vi "Main - 副本.vi"() -> ()   [LabVIEW 2020]
uses:
  System.Windows.Forms
  Global_Variable/Global.vi
  Database/Global1.vi
  <userlib>/_MGI/Menu Building/MenuTypes/MenuStrip/MGI_MenuStrip.lvclass
  <userlib>/_MGI/Menu Building/MenuItemStatusChange/MGI_MenuItemStatusChange.lvclass
  Libraries/S7/S7.lvlib
panel:
  in  "表格控件 2":string[][](table)
  out "上序状态":string
  out "右工位传感器码":string
  in  "表格控件":string[][](table)
  in  "Andon":enum32{"未选择", "缺料报警", "质量报警", "故障报警"}(radio)
  out "PLC":bool
  in  "菜单":refnum<k24>(container)
  out "试验计时":u16
  out "左工位传感器码":string
  out "生产数量":i32
  out "合格数量":i32
  out "userStatus":string caption="用户状态"
  out "userName":string caption="用户名"
  out "connectionMode":string caption="联机类型"
  out "产品型号":string
  in  "更换产品":refnum<vi>
  out "提示信息":string
  out "错误":bool
  out "时间字符串":string
  out "日期字符串":string
  out "自动":bool
  # "芯轴分总成磨合台"
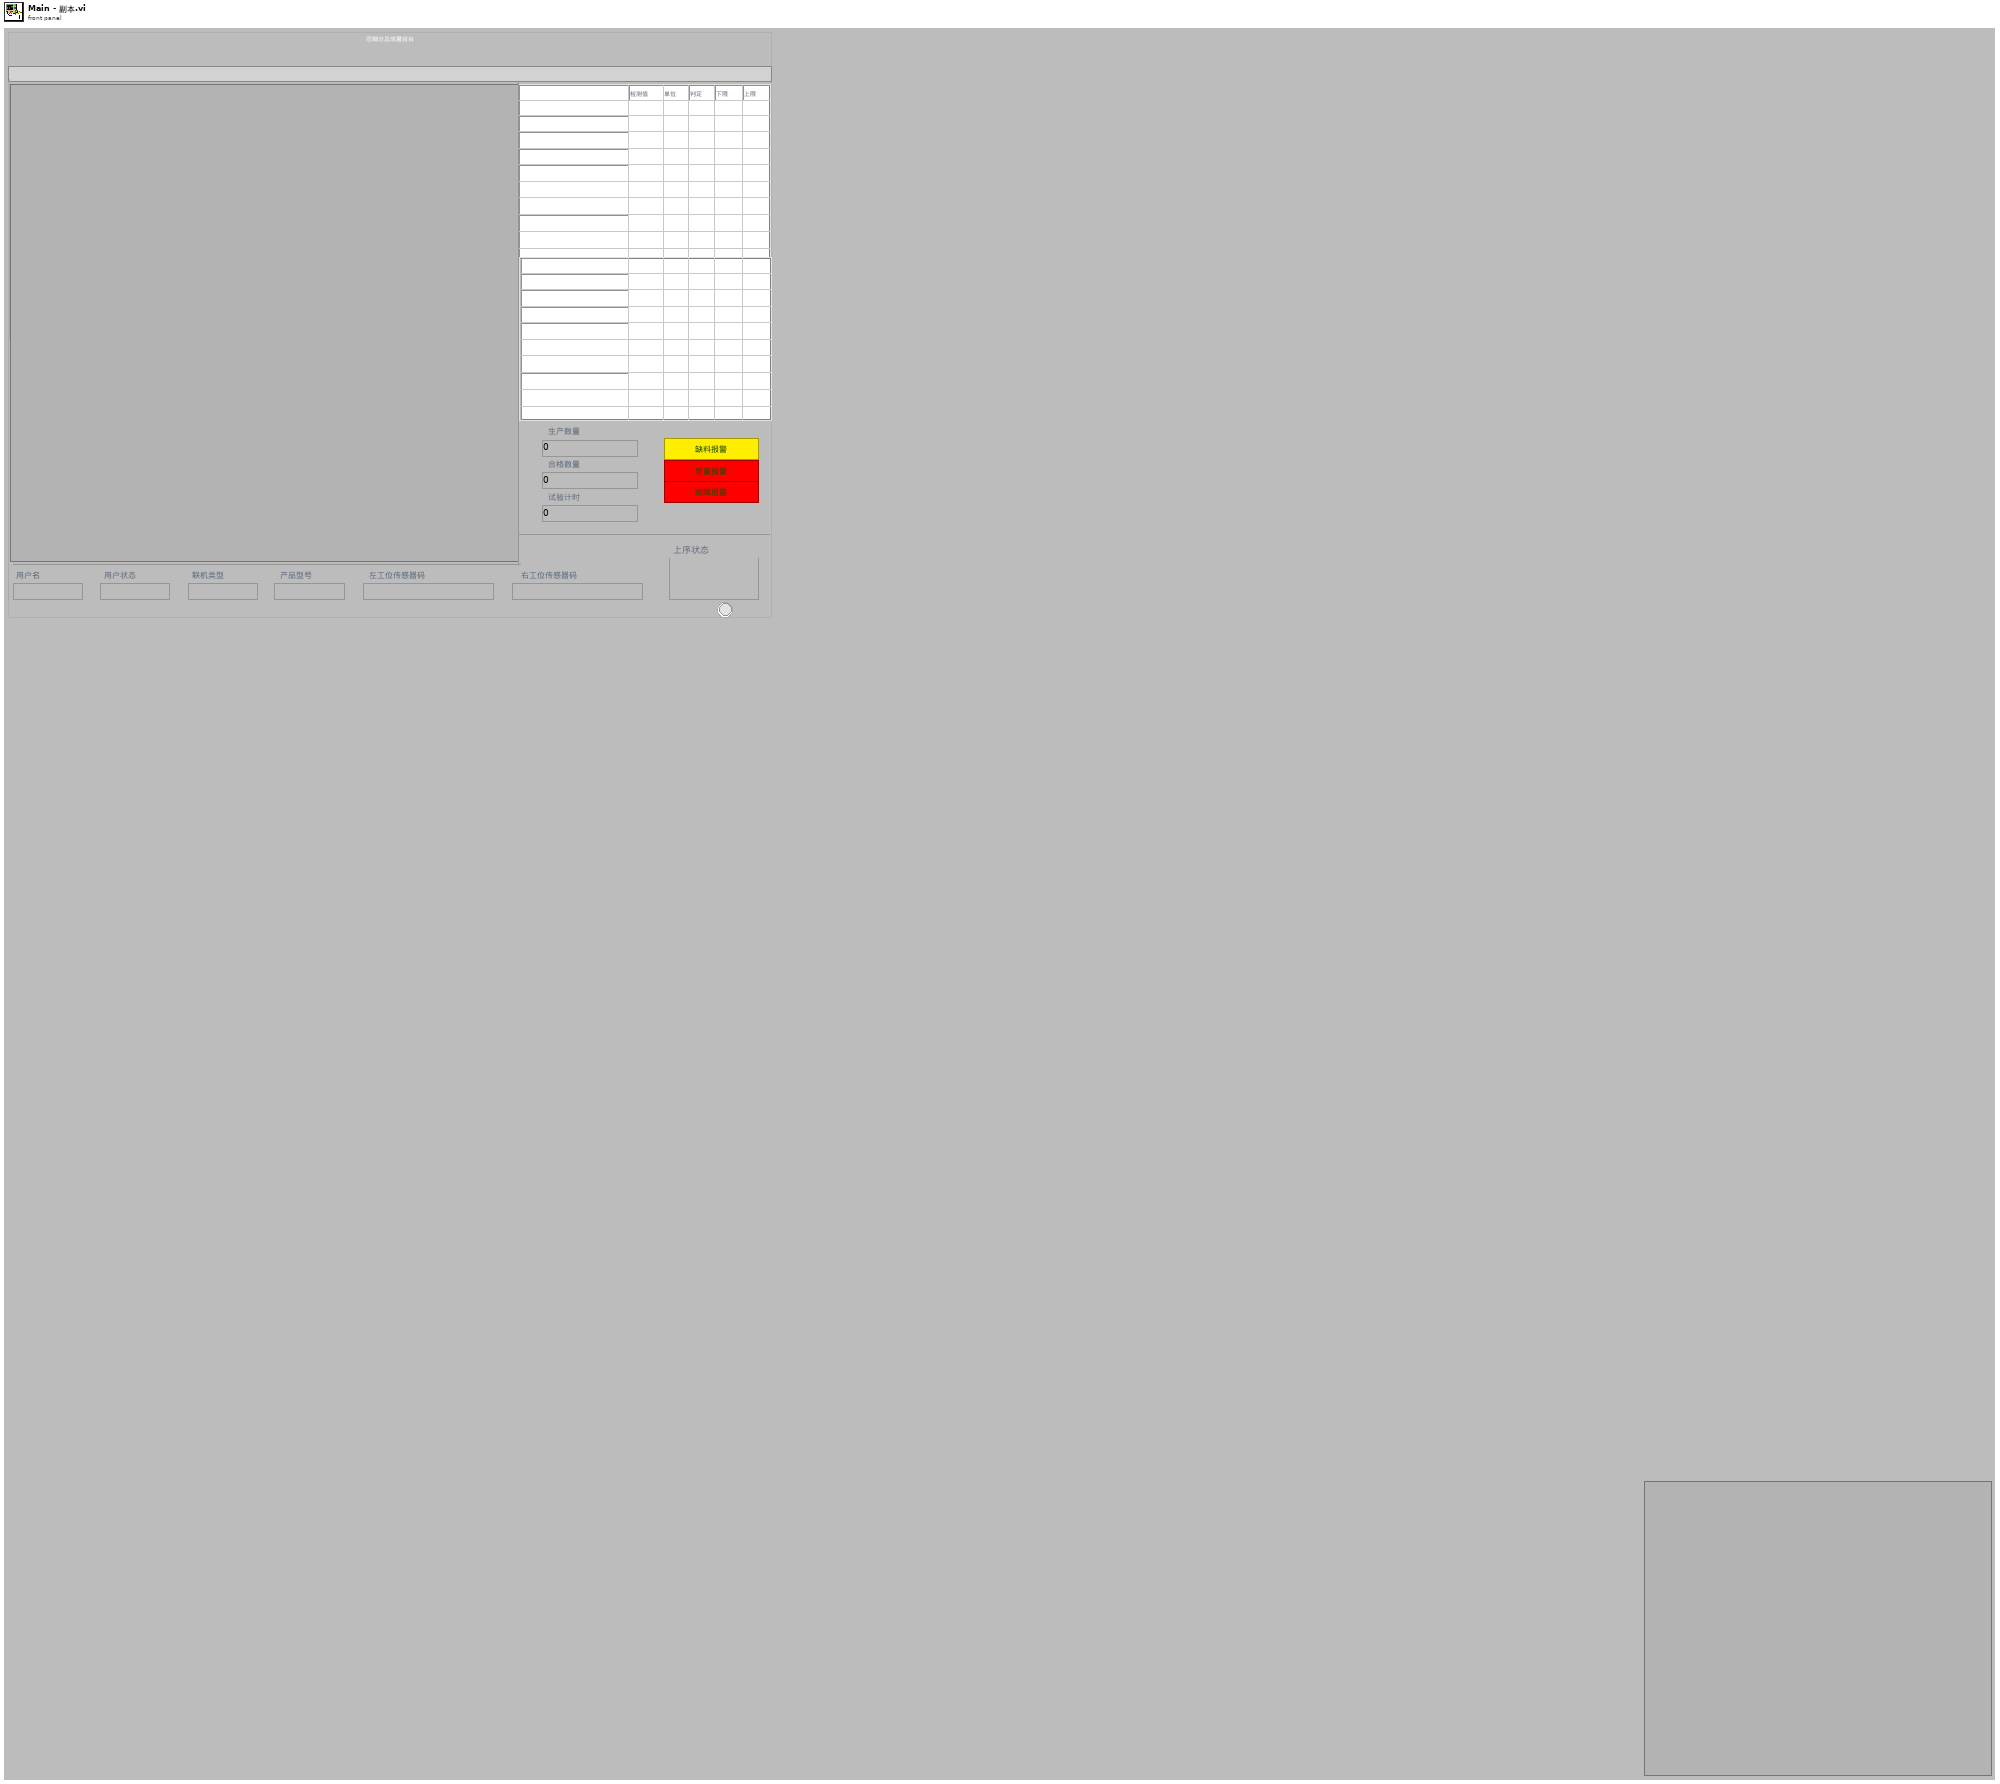
[diagram p1: front panel]
types:
  T1 = typedef "S7.lvlib/Broadcast Events--cluster.ctl" = cluster{"Module Did Init":refnum<user-event>, "Status Updated":refnum<user-event>, "Error Reported":refnum<user-event>, "Module Did Stop":refnum<user-event>, "Update Module Execution Status":refnum<user-event>}
  T2 = enum32{"Invalid", "Standard", "Closed", "Hidden", "Minimized", "Maximized"}
  T3 = cluster{"设备名称":string, "操作人员":string, "设备状态":enum16{"设备离线", "设备正常", "设备缺料", "设备故障", "质量报警"}, "附加信息":string}
  T4 = enum32{"invalid app kind", "Development System", "Run Time System", "Student Edition", "Embedded LabVIEW", "Evaluation", "Custom"}
  T5 = cluster{"用户编号":string, "用户名":string, "用户密码(密文)":string, "用户权限":string}
  T6 = cluster{"Core":cluster{"Current VI Reference":refnum<vi>, "Close Panel on Exit?":bool}, "Your Boolean data":bool, "Your string data":string}
  T7 = cluster{"Current VI Reference":refnum<vi>, "Close Panel on Exit?":bool}
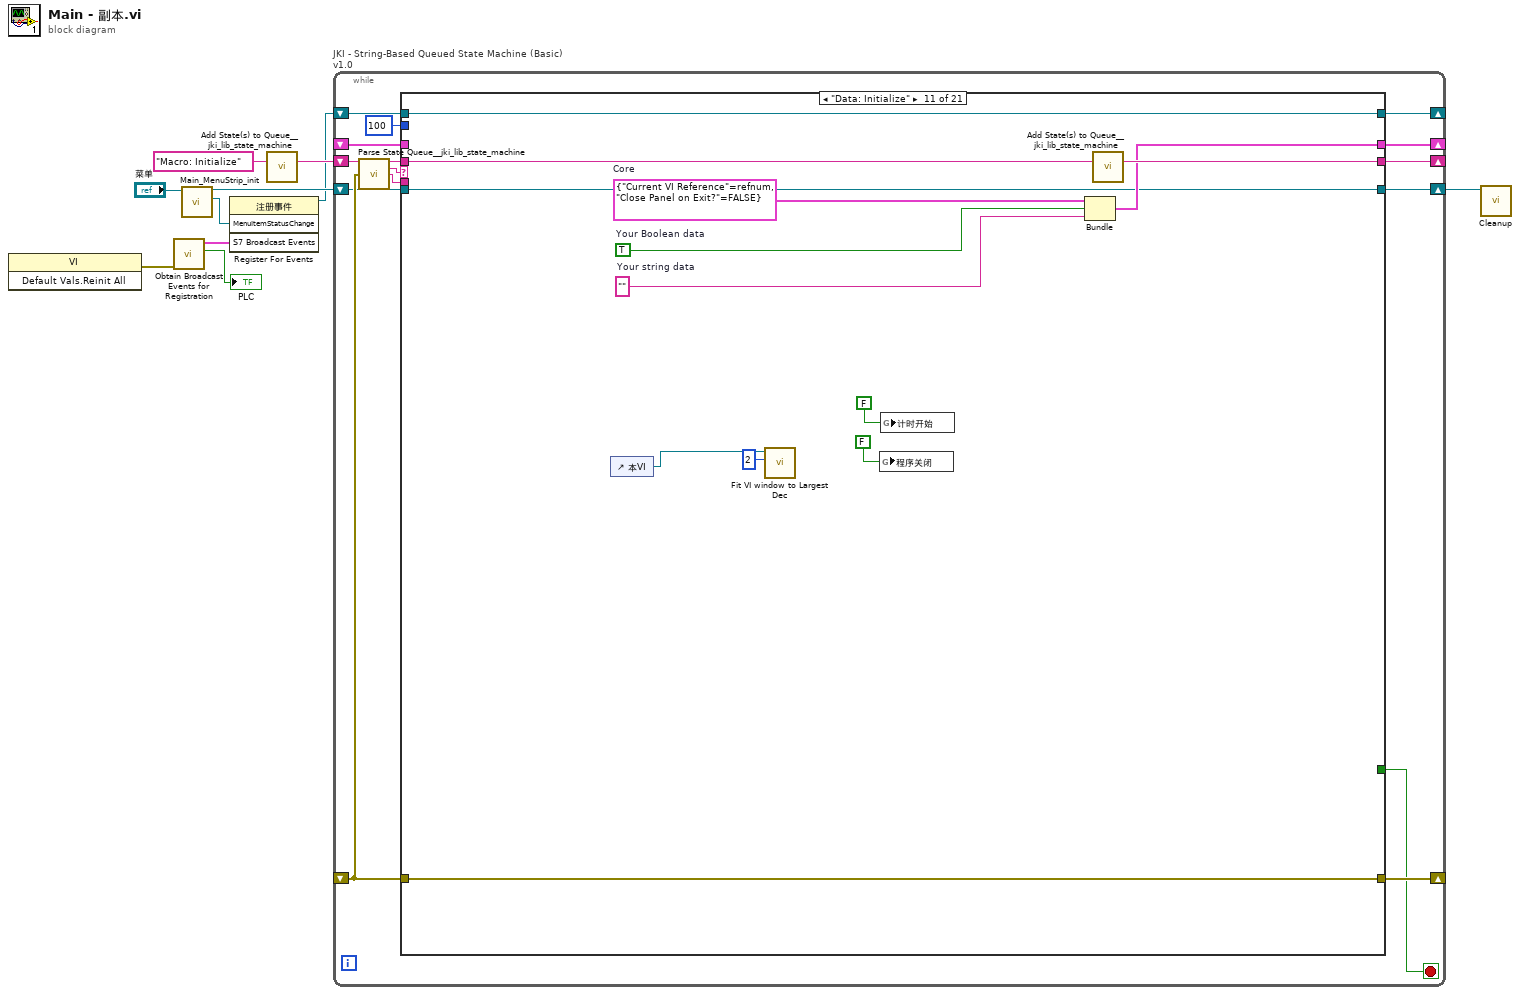
[diagram p0: block diagram]
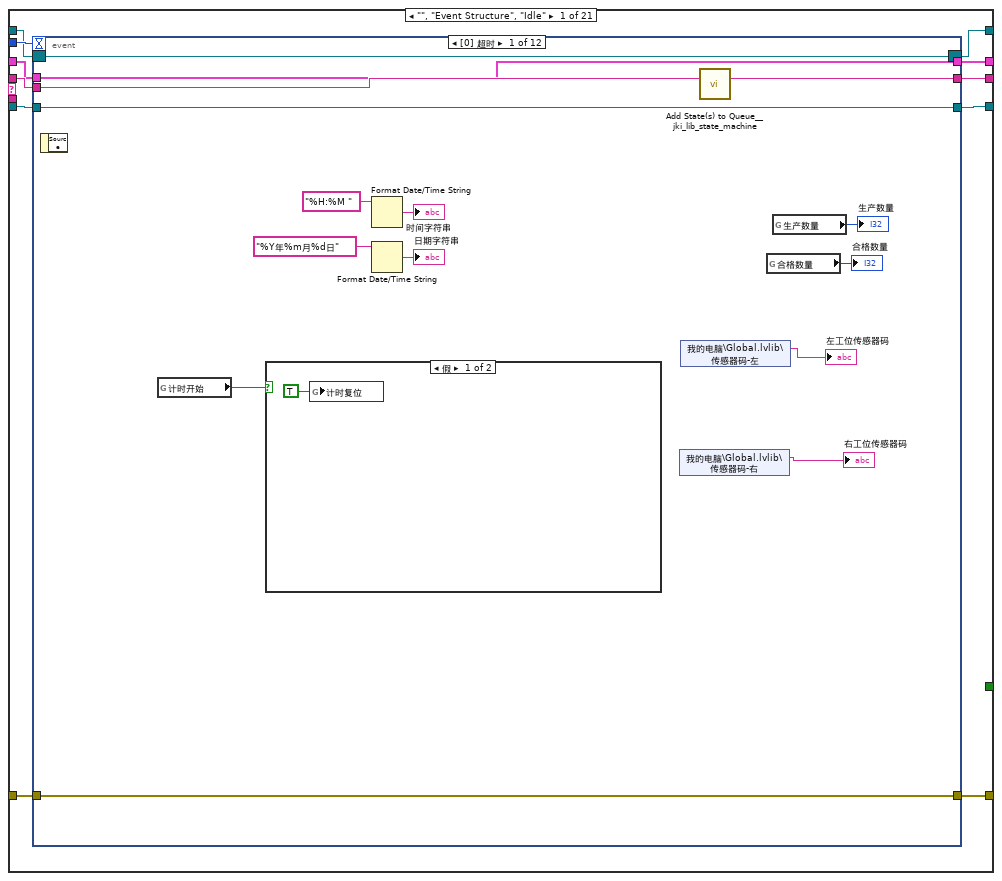
[diagram p2: hidden frame]
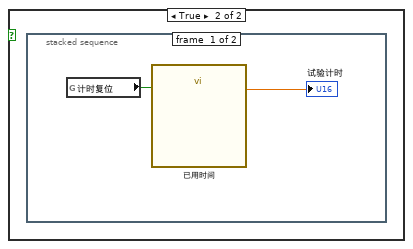
[diagram p3: hidden frame]
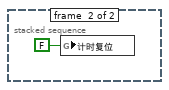
[diagram p4: hidden frame]
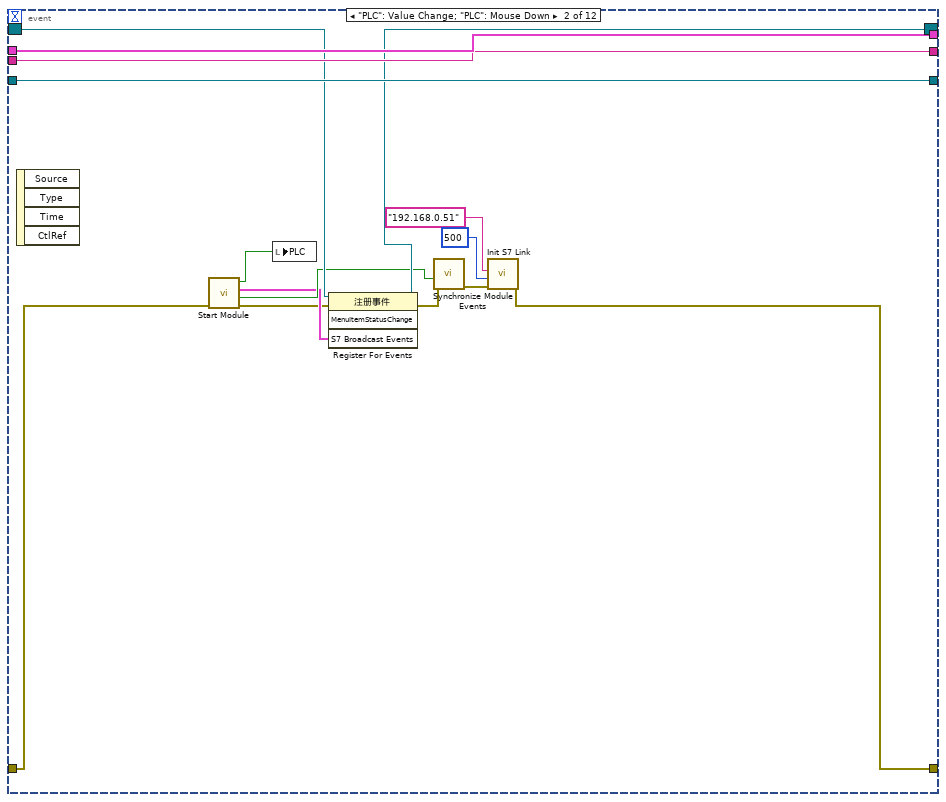
[diagram p5: hidden frame]
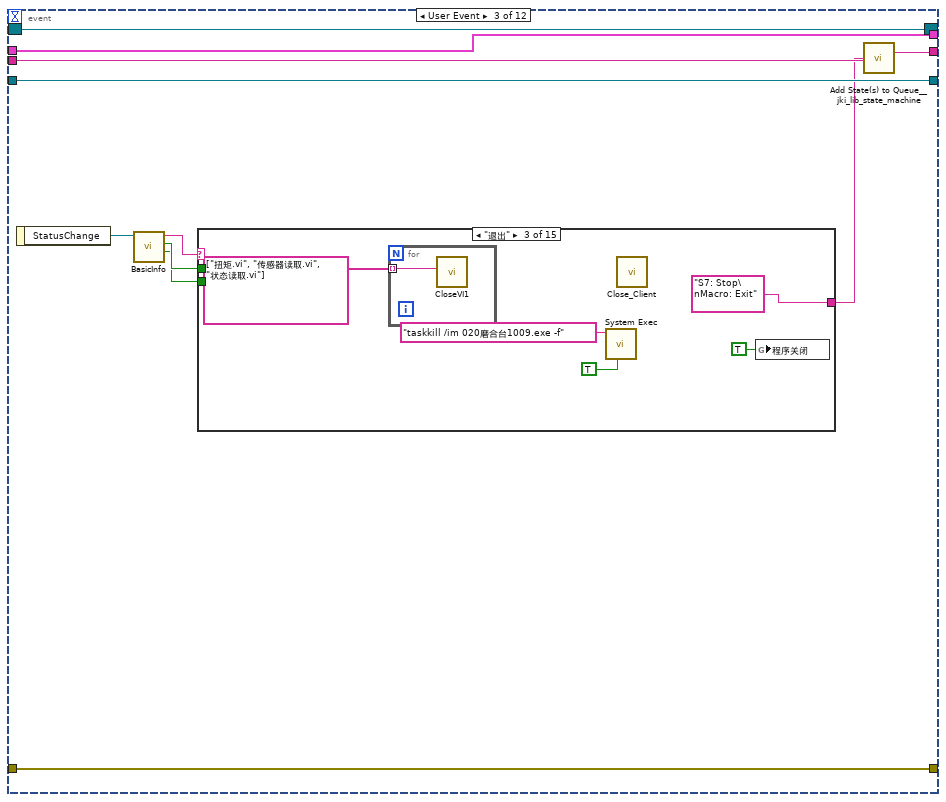
[diagram p6: hidden frame]
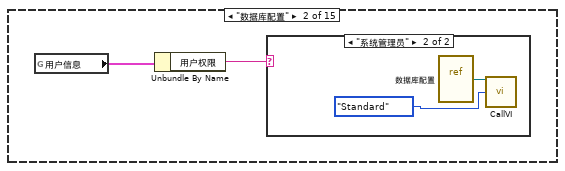
[diagram p8: hidden frame]
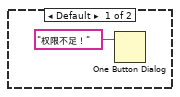
[diagram p9: hidden frame]
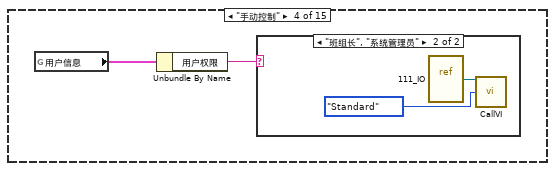
[diagram p10: hidden frame]
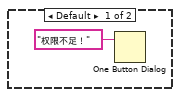
[diagram p11: hidden frame]
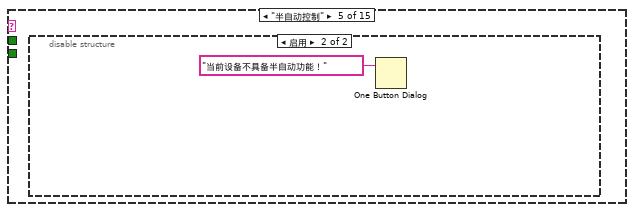
[diagram p12: hidden frame]
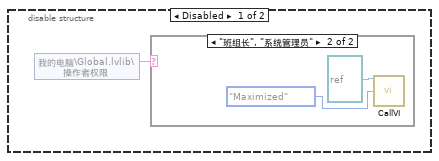
[diagram p13: hidden frame]
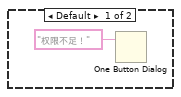
[diagram p14: hidden frame]
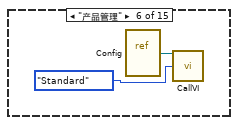
[diagram p15: hidden frame]
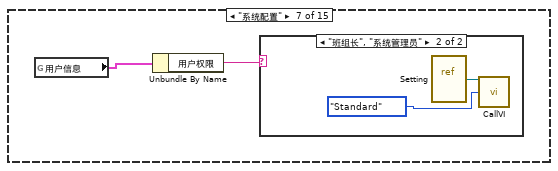
[diagram p16: hidden frame]
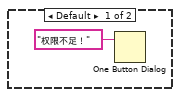
[diagram p17: hidden frame]
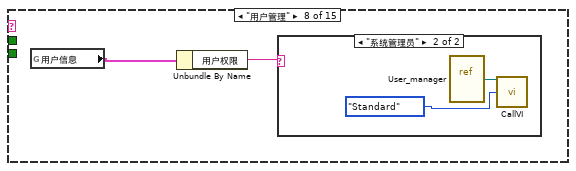
[diagram p18: hidden frame]
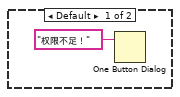
[diagram p19: hidden frame]
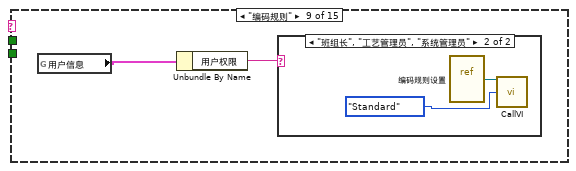
[diagram p20: hidden frame]
diagram:
  n1 = invoke class="VI" method="Default Vals.Reinit All"() -> (error out=w3:errorcluster)  [unwired: 3 in, 2 out]
  n2 = call "Obtain Broadcast Events for Registration.vi"("error in (no error)"=w3) -> ("Already running?"=→"PLC":bool, "S7 Broadcast Events"=w5:T1)  [unwired: 8 in, 1 out]
  n3 = call "Main_MenuStrip_init.vi"("MenuStrip"="菜单") -> ("MenuItemStatusChange"=w2:refnum<user-event>, "Menu out"=w7:refnum<class "MGI_MenuStrip.lvclass">)  [unwired: 9 in]
  n4 = register-events(w2, w5) -> (reference out=w1:refnum<event-registration>)  [unwired: 2 in, 1 out]
  n5 = call <vilib>:"Add State(s) to Queue__jki_lib_state_machine.vi"("State(s) in (\"\")"="Macro: Initialize") -> ("States Out"=w10:string)  [unwired: 14 in]
  n6 = while "JKI - String-Based Queued State Machine (Basic) v1.0" {
    shift-right: [w19] -> _
    shift-left: _ -> [w18]
    shift-right: [w21] -> _
    shift-left: _ -> [w16]
    shift-right: [w20] -> _
    shift-left: w10 -> [w22]
    shift-right: [w14] -> w6
    shift-left: w7 -> [w15]
    shift-right: [w12] -> _
    shift-left: w1 -> [w11]
    stop <- w13 stop-if-true
    n7 = call <vilib>:"Parse State Queue__jki_lib_state_machine.vi"("State Queue"=w22, "Error In (no error)"=w16) -> ("Remaining States"=w24:string, "Current State"=w25:string, "Arguments"=w23:string)  [unwired: 11 in]
    n8 = case shown="\"Data: Initialize\"" w25 {
      selector: w25 -> [_ _ w234 _ _ _ _ _ _ _ _ _ _ _ _ _ _ _ _ _ _]
      tunnel: w24 -> [w36 w231 w238 w258 w266 w274 w280 w284 w290 w299 w312 w320 w326 w339 w363 w400 w408 w421 w449 w456 w468]
      tunnel: w23 -> [_ _ _ _ _ _ _ _ _ _ _ _ _ _ _ _ w403 w415 _ _ _]
      tunnel: w18 -> [w34 w228 w236 w249 w263 w272 w277 w285 w293 w296 _ w315 w323 w337 w361 w397 w406 w417 w446 w453 w465]
      tunnel: [w33 w229 w240 w255 errorcluster {"status"=FALSE, "code"=0, "source"=""} ("error out") w271 w278 w282 w288 w297 w309 w316 w324 w336 w359 w398 w404 w418 w447 w454 w466] -> w21
      tunnel: w16 -> [w32 w229 w239 w255 w262 w271 w278 w282 w289 w297 w309 w317 w324 w333 w359 w398 w405 w419 w447 w454 w466]
      tunnel: [w35 w230 w237 w257 w265 w273 w279 w284 w291 w298 w311 w319 w325 w338 w362 w399 w407 w420 w448 w455 w467] -> w20
      tunnel: [w31 w228 w236 w256 w263 w272 w277 w285 w293 w296 w310 w315 w323 w337 w361 w397 w406 w417 w446 w453 w465] -> w19
      tunnel: 100 ("Timeout") -> [w30 _ _ _ _ _ _ _ _ _ _ _ _ _ _ _ _ _ _ _ _]
      tunnel: w15 -> [w29 w227 w233 w246 w260 w270 w276 w283 w292 w295 w304 w314 w322 w335 w360 w396 w402 w414 w445 w451 w458]
      tunnel: [w28 w227 w233 w246 w260 w270 w276 w283 w292 w295 w304 w314 w322 w335 w360 w396 w402 w414 w445 w451 w458] -> w14
      tunnel: [_ _ _ _ _ TRUE _ _ _ _ _ _ _ _ _ _ _ _ _ _ _] -> w13
      tunnel: [w26 w226 w232 w245 w259 w268 w275 w286 w287 w294 w305 w313 w321 w334 w358 w393 w401 w413 w444 w450 w457] -> w12
      tunnel: w11 -> [w27 w226 w232 w245 w259 w268 w275 w286 w287 w294 w305 w313 w321 w334 w358 w393 w401 w413 w444 w450 w457]
      frame "", "Event Structure", "Idle" {
        n9 = event shown="[0] 超时" {
          selector: w27 -> [w41 w65 w71 w141 w148 w155 w162 w176 w185 w193 w202 _]
          dyn-events: [w41 w64 w71 w141 w148 w155 w162 w176 w185 w193 w202 _] -> w26
          timeout: w30 -> [_ _ _ _ _ _ _ _ _ _ _ _]
          tunnel: w36 -> [w51 w69 w80 w142 w149 w158 w165 w173 w189 w200 w204 w220]
          tunnel: [w50 w69 w78 w143 w150 w159 w166 w174 w190 w199 w205 w220] -> w35
          tunnel: w34 -> [w49 w70 w79 w145 w153 w160 w167 w175 w191 w197 w207 w221]
          tunnel: [w42 w66 w81 w146 w151 w156 w168 w171 w188 w198 w206 w218] -> w33
          tunnel: w32 -> [w42 w67 w81 w146 w151 w156 w169 w171 w188 w198 w206 w218]
          tunnel: [w49 w70 w79 w145 w153 w160 w167 w175 w191 w197 w207 w221] -> w31
          tunnel: w29 -> [w40 w68 w74 w144 w152 w157 w164 w172 _ _ _ w219]
          tunnel: [w40 w68 w74 w144 w152 w157 w164 w172 _ _ _ w219] -> w28
          event Timeout {
            n10 = event-data() -> ()  [unwired: 1 in, 1 out]
            n11 = global read "Global.vi" "计时开始"() -> (w39:bool)
            n12 = case shown="假" w39 {
              frame False {
                n13 = global write "Global.vi" "计时复位"(TRUE ("计时复位")) -> ()
              }
              frame True {
                n14 = stacked-sequence {
                  frame #0 {
                    n15 = global read "Global.vi" "计时复位"() -> (w53:bool)
                    n16 = call "已用时间"("Reset"=w53) -> ("Elapsed Time (s)"=→"试验计时":dbl)  [unwired: 11 in, 7 out]
                  }
                  frame #1 {
                    n17 = global write "Global.vi" "计时复位"(FALSE ("计时复位")) -> ()
                  }
                }
              }
            }
            n18 = Format Date/Time String(time format string (%c)="%H:%M ") -> (date/time string=→"时间字符串":string)  [unwired: 2 in]
            n19 = Format Date/Time String(time format string (%c)="%Y年%m月%d日") -> (date/time string=→"日期字符串":string)  [unwired: 2 in]
            n20 = shared-variable "我的电脑\\Global.lvlib\\传感器码-右"() -> (→"右工位传感器码":string)  [unwired: 1 in, 1 out]
            n21 = shared-variable "我的电脑\\Global.lvlib\\传感器码-左"() -> (→"左工位传感器码":string)  [unwired: 1 in, 1 out]
            n22 = call <vilib>:"Add State(s) to Queue__jki_lib_state_machine.vi"("State(s) in (\"\")"=w51) -> ("States Out"=w50:string)  [unwired: 14 in]
            n23 = global read "Global.vi" "合格数量"() -> (→"合格数量":i32)
            n24 = global read "Global.vi" "生产数量"() -> (→"生产数量":i32)
          }
          event "PLC": Value Change; "PLC": Mouse Down {
            n25 = event-data() -> ()  [unwired: 1 in, 4 out]
            n26 = call "Start Module.vi"("error in (no error)"=w67) -> ("error out"=w60:errorcluster, "Wait for Event Sync?"=w63:bool, "S7 Broadcast Events"=w62:T1, "Module Was Already Running?"=w61:bool)  [unwired: 7 in]
            n27 = local write "PLC"(w61) -> ()
            n28 = register-events(reference=w65, error in=w60, w62) -> (reference out=w64:refnum<event-registration>, error out=w59:errorcluster)  [unwired: 1 in]
            n29 = call "Synchronize Module Events.vi"("error in (no error)"=w59, "Wait for Event Sync?"=w63) -> ("error out"=w56:errorcluster)  [unwired: 9 in]
            n30 = call "Init S7 Link.vi"("error in (no error)"=w56, "超时"=500, "IP"="192.168.0.51") -> ("error out"=w66:errorcluster)  [unwired: 8 in]
          }
          event User Event {
            n31 = event-data() -> ("StatusChange"=w72:refnum<class "MGI_MenuItemStatusChange.lvclass">)  [unwired: 1 in]
            n32 = call <userlib>:"BasicInfo.vi"("MGI_MenuItemStatusChange in"=w72) -> ("Enabled?"=w75:bool, "Checked?"=w76:bool, "Tag"=w77:string)  [unwired: 7 in, 1 out]
            n33 = case shown="\"退出\"" w77 {
              tunnel: w76 -> [_ _ _ _ _ _ _ _ _ _ _ _ _ _ _]
              tunnel: w75 -> [_ _ _ _ _ _ _ _ _ _ _ _ _ _ _]
              tunnel: [_ _ "S7: Stop\nMacro: Exit" _ _ _ _ _ _ _ _ _ _ _ _] -> w73
              frame "假", Default {
              }
              frame "数据库配置" {
                n34 = global read "Global1.vi" "用户信息"() -> (w82:T5)
                n35 = Unbundle By Name(w82) -> ("用户权限"=w83:string)
                n36 = case shown="\"系统管理员\"" w83 {
                  frame Default {
                    n37 = One Button Dialog(message="权限不足！" ("消息")) -> ()  [unwired: 1 in, 1 out]
                  }
                  frame "系统管理员" {
                    n38 = vi-ref "数据库配置.vi"() -> (w86:refnum<vi>)
                    n39 = call "CallVI.vi"("VI引用"=w86, "状态"=T2."Standard") -> ()  [unwired: 11 in, 3 out]
                  }
                }
              }
              frame "退出" {
                n40 = for {
                  tunnel: string[] ["扭矩.vi", "传感器读取.vi", "状态读取.vi"] -> [w92] mode=indexing
                  n41 = call "CloseVI1.vi"("名称或相对路径"=w92) -> ()  [unwired: 10 in, 1 out]
                }
                n42 = call <vilib>:"System Exec.vi"("run minimized? (F)"=TRUE, "command line"="taskkill /im 020磨合台1009.exe -f") -> ()  [unwired: 6 in, 4 out]
                n43 = call "Close_Client.vi"() -> ()  [unwired: 12 in]
                n44 = global write "Global.vi" "程序关闭"(TRUE ("程序关闭")) -> ()
              }
              frame "手动控制" {
                n45 = global read "Global1.vi" "用户信息"() -> (w93:T5)
                n46 = Unbundle By Name(w93) -> ("用户权限"=w94:string)
                n47 = case shown="\"班组长\", \"系统管理员\"" w94 {
                  frame Default {
                    n48 = One Button Dialog(message="权限不足！" ("消息")) -> ()  [unwired: 1 in, 1 out]
                  }
                  frame "班组长", "系统管理员" {
                    n49 = vi-ref "111_IO.vi"() -> (w97:refnum<vi>)
                    n50 = call "CallVI.vi"("VI引用"=w97, "状态"=T2."Standard") -> ()  [unwired: 11 in, 3 out]
                  }
                }
              }
              frame "半自动控制" {
                n51 = disable-structure shown="启用" {
                  frame Disabled {
                    n52 = shared-variable "我的电脑\\Global.lvlib\\操作者权限"() -> (w98:string)  [unwired: 1 in, 1 out]
                    n53 = case shown="\"班组长\", \"系统管理员\"" w98 {
                      frame Default {
                        n54 = One Button Dialog(message="权限不足！" ("消息")) -> ()  [unwired: 1 in, 1 out]
                      }
                      frame "班组长", "系统管理员" {
                        n55 = call "CallVI.vi"("VI引用"=refnum<vi> refnum, "状态"=T2."Maximized") -> ()  [unwired: 11 in, 3 out]
                      }
                    }
                  }
                  frame Enabled {
                    n56 = One Button Dialog(message="当前设备不具备半自动功能！" ("消息")) -> ()  [unwired: 1 in, 1 out]
                  }
                }
              }
              frame "产品管理" {
                n57 = vi-ref "Config.vi"() -> (w104:refnum<vi>)
                n58 = call "CallVI.vi"("VI引用"=w104, "状态"=T2."Standard") -> ()  [unwired: 11 in, 3 out]
              }
              frame "系统配置" {
                n59 = global read "Global1.vi" "用户信息"() -> (w105:T5)
                n60 = Unbundle By Name(w105) -> ("用户权限"=w106:string)
                n61 = case shown="\"班组长\", \"系统管理员\"" w106 {
                  frame Default {
                    n62 = One Button Dialog(message="权限不足！" ("消息")) -> ()  [unwired: 1 in, 1 out]
                  }
                  frame "班组长", "系统管理员" {
                    n63 = vi-ref "Setting.vi"() -> (w109:refnum<vi>)
                    n64 = call "CallVI.vi"("VI引用"=w109, "状态"=T2."Standard") -> ()  [unwired: 11 in, 3 out]
                  }
                }
              }
              frame "用户管理" {
                n65 = global read "Global1.vi" "用户信息"() -> (w110:T5)
                n66 = Unbundle By Name(w110) -> ("用户权限"=w111:string)
                n67 = case shown="\"系统管理员\"" w111 {
                  frame Default {
                    n68 = One Button Dialog(message="权限不足！" ("消息")) -> ()  [unwired: 1 in, 1 out]
                  }
                  frame "系统管理员" {
                    n69 = vi-ref "User_manager.vi"() -> (w114:refnum<vi>)
                    n70 = call "CallVI.vi"("VI引用"=w114, "状态"=T2."Standard") -> ()  [unwired: 11 in, 3 out]
                  }
                }
              }
              frame "编码规则" {
                n71 = global read "Global1.vi" "用户信息"() -> (w115:T5)
                n72 = Unbundle By Name(w115) -> ("用户权限"=w116:string)
                n73 = case shown="\"班组长\", \"工艺管理员\", \"系统管理员\"" w116 {
                  frame Default {
                    n74 = One Button Dialog(message="权限不足！" ("消息")) -> ()  [unwired: 1 in, 1 out]
                  }
                  frame "班组长", "工艺管理员", "系统管理员" {
                    n75 = vi-ref "编码规则设置.vi"() -> (w119:refnum<vi>)
                    n76 = call "CallVI.vi"("VI引用"=w119, "状态"=T2."Standard") -> ()  [unwired: 11 in, 3 out]
                  }
                }
              }
              frame "易损件管理" {
                n77 = vi-ref "易损件管理.vi"() -> (w121:refnum<vi>)
                n78 = call "CallVI.vi"("VI引用"=w121, "状态"=T2."Standard") -> ()  [unwired: 11 in, 3 out]
              }
              frame "物料批次管理" {
                n79 = vi-ref "批次管理.vi"() -> (w123:refnum<vi>)
                n80 = call "CallVI.vi"("VI引用"=w123, "状态"=T2."Standard") -> ()  [unwired: 11 in, 3 out]
              }
              frame "报表" {
                n81 = call "文件对话框"("start path"=path "D:/report", "prompt"="打开报表", "pattern (all files)"="*.doc;*.docx", "pattern label"="Word 文档") -> ("selected path"=w124:path, "error out"=w125:errorcluster)  [unwired: 8 in, 2 out]
                n82 = case shown="无错误" w125 {
                  selector: w125 -> [w131 w133]
                  tunnel: w124 -> [w132 _]
                  frame No Error {
                    w130 = 1 items=["Normal", "Maximize", "Minimize"] ("cpubbs_WindowState")
                    n83 = call "Open_Word.vi"("File Path"=w132, "cpubbs_WindowState"=w130, "错误输入（无错误）"=w131) -> ()  [unwired: 12 in, 1 out]
                  }
                  frame Error {
                    n84 = call <vilib>:"Clear Errors.vi"("error in (no error)"=w133) -> ()  [unwired: 5 in, 2 out]
                  }
                }
              }
              frame "报警信息" {
                n85 = vi-ref "报警信息.vi"() -> (w135:refnum<vi>)
                n86 = call "CallVI.vi"("VI引用"=w135, "状态"=T2."Standard") -> ()  [unwired: 11 in, 3 out]
              }
              frame "关于" {
                n87 = vi-ref "About.vi"() -> (w137:refnum<vi>)
                n88 = call "CallVI.vi"("VI引用"=w137, "状态"=T2."Standard") -> ()  [unwired: 11 in, 3 out]
              }
              frame "操作演示" {
                n89 = call <vilib>:"Application Directory.vi"() -> ("Application Directory"=w140:path)
                n90 = Build Path(base path=w140, name or relative path="操作演示" ("名称或相对路径")) -> (appended path=w139:path)
                n91 = call "自动播放ppt.vi"("路径"=w139) -> ()  [unwired: 10 in, 1 out]
              }
            }
            n92 = call <vilib>:"Add State(s) to Queue__jki_lib_state_machine.vi"("State(s) in (\"\")"=w80, "State(s) at Back (\"\")"=w73) -> ("States Out"=w78:string)  [unwired: 13 in]
          }
          event User Event {
            n93 = event-data() -> ("Init?"=w147:bool)  [unwired: 1 in, 1 out]
            n94 = local write "PLC"(w147) -> ()
            n95 = call <vilib>:"Add State(s) to Queue__jki_lib_state_machine.vi"("State(s) in (\"\")"=w142) -> ("States Out"=w143:string)  [unwired: 14 in]
          }
          event User Event {
            n96 = event-data() -> ("Running?"=w154:bool)  [unwired: 1 in]
            n97 = local write "PLC"(w154) -> ()
            n98 = call <vilib>:"Add State(s) to Queue__jki_lib_state_machine.vi"("State(s) in (\"\")"=w149) -> ("States Out"=w150:string)  [unwired: 14 in]
          }
          event User Event {
            n99 = event-data() -> ()  [unwired: 1 in, 7 out]
            n100 = local write "PLC"(FALSE ("PLC")) -> ()
            n101 = call <vilib>:"Add State(s) to Queue__jki_lib_state_machine.vi"("State(s) in (\"\")"=w158) -> ("States Out"=w159:string)  [unwired: 14 in]
          }
          event User Event {
            n102 = event-data() -> ("Error"=w170:errorcluster)  [unwired: 1 in]
            n103 = Merge Errors(w170, w169) -> (w168:errorcluster)
            n104 = call <vilib>:"Add State(s) to Queue__jki_lib_state_machine.vi"("State(s) in Front (\"\")"="S7: Initialize\nIdle", "State(s) in (\"\")"=w165) -> ("States Out"=w166:string)  [unwired: 13 in]
          }
          event "自动": Mouse Down {
            n105 = event-data() -> ()  [unwired: 1 in, 1 out]
            n106 = disable-structure shown="禁用" {
              frame Disabled {
                n107 = local read "自动"() -> (w177:bool)
                n108 = case shown="假" w177 {
                  frame False {
                    n109 = call "设备状态.vi"() -> ("Status_Read"=w178:i16)  [unwired: 11 in]
                    n110 = case shown="5" w178 {
                      frame 0, Default {
                        n111 = One Button Dialog(message="请复位！" ("消息")) -> ()  [unwired: 1 in, 1 out]
                      }
                      frame 5 {
                      }
                    }
                  }
                  frame True {
                    n112 = Two Button Dialog(message="确定要退出自动？" ("消息")) -> (T button?=w180:bool)  [unwired: 2 in]
                    n113 = case shown="真" w180 {
                      frame False {
                      }
                      frame True {
                        n114 = vi-ref "Auto - 副本.vi"() -> (w184:refnum<vi>)
                        n115 = invoke class="VI" method="Ctrl Val.Set"(reference=w184, "Control Name"="STEP" ("控件名"), "Value"="退出自动" ("控件名")) -> ()  [unwired: 2 in, 5 out]
                      }
                    }
                  }
                }
              }
              frame Enabled {
              }
            }
            n116 = call <vilib>:"Add State(s) to Queue__jki_lib_state_machine.vi"("State(s) in (\"\")"=w173) -> ("States Out"=w174:string)  [unwired: 14 in]
          }
          event "错误": Mouse Down {
            n117 = event-data() -> ()  [unwired: 1 in, 8 out]
            n118 = vi-ref "报警信息.vi"() -> (w187:refnum<vi>)
            n119 = call "CallVI.vi"("VI引用"=w187, "状态"=T2."Standard") -> ()  [unwired: 11 in, 3 out]
            n120 = call <vilib>:"Add State(s) to Queue__jki_lib_state_machine.vi"("State(s) in (\"\")"=w189) -> ("States Out"=w190:string)  [unwired: 14 in]
          }
          event Panel Close? {
            n121 = event-data() -> ()  [unwired: 1 in, 1 out]
            n122 = global write "Global.vi" "计时开始"(FALSE ("计时复位")) -> ()
            n123 = global write "Global.vi" "程序关闭"(TRUE ("程序关闭")) -> ()
            n124 = call <vilib>:"Add State(s) to Queue__jki_lib_state_machine.vi"("State(s) in Front (\"\")"="S7: Stop\nMacro: Exit", "State(s) in (\"\")"=w200) -> ("States Out"=w199:string)  [unwired: 13 in]
            n125 = event-data("Discard?"=TRUE) -> ()  [unwired: 1 in, 1 out]
          }
          event "更换产品": Value Change {
            n126 = event-data() -> ("NewVal"=w203:refnum<vi>)  [unwired: 1 in, 5 out]
            n127 = stacked-sequence {
              tunnel: w203 -> [w210]
              tunnel: ["Idle"] -> w201
              frame #0 {
                n128 = disable-structure shown="禁用" {
                  disable-tunnel: w210 -> [w212 _]
                  frame Disabled {
                    n129 = control-ref of="子面板"() -> (w211:refnum<vi>)
                    n130 = call "Call_SubPanal.vi"("VI引用句柄"=w212, "SubPnl引用句柄"=w211) -> ()  [unwired: 9 in, 1 out]
                  }
                  frame Enabled {
                  }
                }
                n131 = shared-variable "我的电脑\\Global.lvlib\\产品型号"() -> (w209:string)  [unwired: 1 in, 1 out]
                n132 = local write "产品型号"(w209) -> ()
              }
            }
            n133 = call <vilib>:"Add State(s) to Queue__jki_lib_state_machine.vi"("State(s) in Front (\"\")"=w201, "State(s) in (\"\")"=w204) -> ("States Out"=w205:string)  [unwired: 13 in]
          }
          event "Andon": Value Change {
            n134 = event-data() -> ("NewVal"=w217:enum32{"未选择", "缺料报警", "质量报警", "故障报警"})  [unwired: 1 in]
            n135 = case shown="\"故障报警\"" w217 {
              tunnel: [enum16{"设备离线", "设备正常", "设备缺料", "设备故障", "质量报警"}."设备正常" ("设备状态") enum16{"设备离线", "设备正常", "设备缺料", "设备故障", "质量报警"}."设备缺料" ("设备状态") enum16{"设备离线", "设备正常", "设备缺料", "设备故障", "质量报警"}."质量报警" ("设备状态") enum16{"设备离线", "设备正常", "设备缺料", "设备故障", "质量报警"}."设备故障" ("设备状态")] -> w215
              frame "未选择", Default {
              }
              frame "缺料报警" {
              }
              frame "质量报警" {
              }
              frame "故障报警" {
              }
            }
            n136 = local read "userName"() -> (w214:string)
            n137 = Bundle By Name(cluster=T3 {"设备名称"="芯轴分总成磨合台", "操作人员"="", "设备状态"=enum."设备离线", "附加信息"=""} ("设备信息"), "操作人员"=w214, "设备状态"=w215) -> (w213:T3)
            n138 = call "Change_Client.vi"("设备信息"=w213) -> ()  [unwired: 10 in, 1 out]
          }
        }
      }
      frame "---------- Core ----------" {
        n139 = call <vilib>:"Add State(s) to Queue__jki_lib_state_machine.vi"("State(s) in (\"\")"=w231) -> ("States Out"=w230:string)  [unwired: 14 in]
      }
      frame Default {
        w243 = 42 items=["No error", "Argument error", "Memory is full", "Out of zone", "End of file", "File already open", "Generic file I/O error", "File not found", "File permission error", "Disk is full", "Duplicate path", "Too many files open", "System feature not enabled", "Resource file not found", "Cannot add resource", "Resource not found", "Image not found", "Image memory error", "Pen does not exist", "Config type invalid", "Config token not found", "Config parse error", "Config memory error", "Bad external code format", "Bad external code offset", "External code not present", "Null window", "Destroy window error", "Null menu", "Print aborted", "Bad print record", "Print driver error", "Windows error during printing", "Memory error during printing", "Print dialog error", "Generic print error", "Invalid device refnum", "Device not found", "Device parameter error", "Device unit error", "Cannot open device", "Device call aborted", "Generic error", "Cancelled by user", "Object ID too low", "Object ID too high", "Object not in heap", "Unknown heap", "Unknown object (invalid DefProc)", "Unknown object (DefProc not in table)", "Message out of range", "Invalid (null) method", "Unknown message", "Manager call not supported", "Bad address", "Network operation in progress", "Network operation timed out", "Connection is busy", "Network attribute not supported", "Network error", "Address in use", "System out of memory", "Connection aborted", "Connection refused", "Not connected", "Already connected", "Connection closed", "Initialization error (interapplication manager)", "Bad occurrence", "Wait on unbound occurrence handler", "Occurrence queue overflow", "Datalog type conflict", "Unused", "Unrecognized type (interapplication manager)", "Memory corrupt", "Failed to make temporary DLL", "Old CIN version", "Drag socket not found", "Failed to load drop-object", "Failed to register OLE object", "Failed to release OLE object", "Format specifier type mismatch", "Unknown format specifier", "Too few format specifiers", "Too many format specifiers", "Scan failed", "Newer CIN version", "Error converting to variant", "Runtime menu error", "Password tampered", "Variant attribute not found", "Incompatible variant data type", "Event data is not available", "Event Store is not present", "Occurrence is not found", "Event Queue is not created", "Event info is not available", "Refnum passed is NULL", "Error retrieving Class GUID", "Error retrieving CoClass GUID", "Error retrieving TypeLib GUID.", "Bad built application magic bytes.", "Specific driver is different from the specific driver associated with the Logical Name.", "There is no session opened to the class driver.", "Max Error", "MAX - Error with config objects", "MAX - Error loading configuration", "MAX - Group not supported"]
        # "Current State"
        n140 = Format Into String(format string="Software Exception: Unhandled State \"%s\"." ("message"), error in=w239, w234) -> (resulting string=w242:string, error out=w241:errorcluster)  [unwired: 1 in]
        n141 = call <vilib>:"Error Cluster From Error Code.vi"("show call chain? (False)"=TRUE, "error in (no error)"=w241, "error message (\"\")"=w242, "error code (0)"=w243) -> ("error out"=w240:errorcluster)  [unwired: 5 in]
        n142 = call <vilib>:"Add State(s) to Queue__jki_lib_state_machine.vi"("State(s) in (\"\")"=w238) -> ("States Out"=w237:string)  [unwired: 14 in]
      }
      frame "Initialize Core Data" {
        # "originally closed?"
        # "exe?"
        n143 = property class="VI"() -> ("Front Panel.Open"=w254:bool)  [unwired: 2 in, 2 out]
        n144 = property class="App"() -> ("App.Kind"=w253:T4)  [unwired: 2 in, 2 out]
        n145 = control-ref of="Current VI Reference"() -> (w247:refnum<vi>)
        n146 = Not(x=w254) -> (.not. x?=w251:bool)
        n147 = Equal?(x=w253, y=T4."Run Time System" ("Application:Kind")) -> (x = y?=w250:bool)
        n148 = Or(x=w251, y=w250) -> (x .or. y?=w248:bool)
        n149 = Bundle By Name(cluster=w249, "Core.Current VI Reference"=w247, "Core.Close Panel on Exit?"=w248) -> (w256:T6)
        n150 = call <vilib>:"Add State(s) to Queue__jki_lib_state_machine.vi"("State(s) in (\"\")"=w258) -> ("States Out"=w257:string)  [unwired: 14 in]
      }
      frame "Error Handler" {
        n151 = call <vilib>:"General Error Handler.vi"("error in (no error)"=w262) -> ()  [unwired: 10 in, 5 out]
        n152 = call <vilib>:"Add State(s) to Queue__jki_lib_state_machine.vi"("State(s) in Front (\"\")"="/* Post Error States", "State(s) in (\"\")"=w266) -> ("States Out"=w265:string)  [unwired: 13 in]
      }
      frame "Exit" {
        n153 = call <vilib>:"Add State(s) to Queue__jki_lib_state_machine.vi"("State(s) in (\"\")"=w274) -> ("States Out"=w273:string)  [unwired: 14 in]
        n154 = Quit LabVIEW(quit? (T)=TRUE ("退出？(T)")) -> ()
      }
      frame "--------- Library --------" {
        n155 = call <vilib>:"Add State(s) to Queue__jki_lib_state_machine.vi"("State(s) in (\"\")"=w280) -> ("States Out"=w279:string)  [unwired: 14 in]
      }
      frame "S7: Initialize" {
        n156 = property on="PLC" class="Bool (严格)"("Val(Sgnl)"=FALSE ("值(信号)")) -> ()  [unwired: 2 in, 2 out]
      }
      frame "S7: Stop" {
        n157 = call "Stop Module.vi"("error in (no error)"=w289) -> ("error out"=w288:errorcluster)  [unwired: 10 in]
        n158 = call <vilib>:"Add State(s) to Queue__jki_lib_state_machine.vi"("State(s) in (\"\")"=w290) -> ("States Out"=w291:string)  [unwired: 14 in]
      }
      frame "---------- Data ----------" {
        n159 = call <vilib>:"Add State(s) to Queue__jki_lib_state_machine.vi"("State(s) in (\"\")"=w299) -> ("States Out"=w298:string)  [unwired: 14 in]
      }
      frame "Data: Initialize" {
        w306 = T7 {"Current VI Reference"=refnum, "Close Panel on Exit?"=FALSE}  # Core
        w308 = TRUE  # Your Boolean data
        w307 = ""  # Your string data
        n160 = control-ref of="本VI"() -> (w301:refnum<vi>)
        n161 = call "Fit VI window to Largest Dec.vi"("border spacing (2 px)"=2, "VI Ref (calling VI)"=w301) -> ()  [unwired: 4 in, 2 out]
        n162 = global write "Global.vi" "程序关闭"(FALSE ("程序关闭")) -> ()
        n163 = global write "Global.vi" "计时开始"(FALSE ("计时结束")) -> ()
        n164 = Bundle("Core"=w306, "Your Boolean data"=w308, "Your string data"=w307) -> (w310:T6)  [unwired: 1 in]
        n165 = call <vilib>:"Add State(s) to Queue__jki_lib_state_machine.vi"("State(s) in (\"\")"=w312) -> ("States Out"=w311:string)  [unwired: 14 in]
      }
      frame "Data: Cleanup" {
        n166 = Unbundle By Name(w315) -> ("Core.Current VI Reference"=w318:refnum<vi>)
        n167 = Close Reference(reference=w318, error in (no error)=w317) -> (error out=w316:errorcluster)
        n168 = call <vilib>:"Add State(s) to Queue__jki_lib_state_machine.vi"("State(s) in (\"\")"=w320) -> ("States Out"=w319:string)  [unwired: 14 in]
      }
      frame "---------- UI ----------" {
        # "Do not put any code in this frame.\n(It is a separator no-op. You can make a copy of this frame to create a new UI frame)"
        n169 = call <vilib>:"Add State(s) to Queue__jki_lib_state_machine.vi"("State(s) in (\"\")"=w326) -> ("States Out"=w325:string)  [unwired: 14 in]
      }
      frame "UI: Initialize" {
        n170 = vi-ref "Auto - 副本.vi"() -> (w332:refnum<vi>)
        n171 = invoke class="VI" method="Ctrl Val.Set"(reference=w332, "Control Name"="STEP" ("控件名"), "Value"="初始化" ("控件名")) -> (reference out=w329:refnum<vi>)  [unwired: 2 in, 4 out]
        n172 = disable-structure shown="启用" {
          disable-tunnel: [w346 _] -> w336
          disable-tunnel: w333 -> [w344 _]
          frame Enabled {
            n173 = vi-ref "Auto - 副本.vi"() -> (w345:refnum<vi>)
            n174 = property class="VI"(reference=w345) -> (reference out=w343:refnum<vi>, "FP.State"=w342:T2)  [unwired: 1 in, 1 out]
            n175 = case shown="\"Standard\", 默认" w342 {
              tunnel: w344 -> [w352 w354]
              tunnel: w343 -> [w353 w355]
              tunnel: [w351 w355] -> w340
              tunnel: [w350 w354] -> w341
              frame "Standard", Default {
                n176 = invoke class="VI" method="FP.Close"(reference=w353, error in=w352) -> (reference out=w351:refnum<vi>, error out=w350:errorcluster)  [unwired: 1 in, 1 out]
              }
              frame "Invalid", "Closed" {
              }
            }
            n177 = invoke on="子面板" class="SubPnl" method="Insert VI"(error in=w341, "VI Ref"=w340) -> (error out=w349:errorcluster)  [unwired: 2 in, 3 out]
            n178 = invoke class="VI" method="Run VI"(reference=w340, error in=w349, "Wait until done"=FALSE ("结束前等待"), "Auto Dispose Ref"=TRUE ("自动销毁引用")) -> (error out=w346:errorcluster)  [unwired: 1 in, 4 out]
          }
          frame Disabled {
            n179 = vi-ref "Auto - 副本.vi"() -> (w357:refnum<vi>)
            n180 = call "CallVI.vi"("VI引用"=w357, "状态"=T2."Maximized") -> ()  [unwired: 11 in, 3 out]
          }
        }
        n181 = invoke class="VI" method="Ctrl Val.Set"(reference=w329, "Control Name"="STEP2" ("控件名"), "Value"="初始化" ("控件名")) -> ()  [unwired: 2 in, 5 out]
        n182 = call <vilib>:"Add State(s) to Queue__jki_lib_state_machine.vi"("State(s) in (\"\")"=w339) -> ("States Out"=w338:string)  [unwired: 14 in]
      }
      frame "UI: Init" {
        n183 = stacked-sequence {
          tunnel: w359 -> [_ _ _ _]
          frame #0 {
            n184 = global write "Global.vi" "程序关闭"(FALSE ("程序关闭")) -> ()
            n185 = vi-ref "状态读取.vi"() -> (w368:refnum<vi>)
            n186 = vi-ref "扭矩.vi"() -> (w367:refnum<vi>)
            n187 = call "CallVI.vi"("VI引用"=w368, "状态"=T2."Hidden") -> ("错误输出"=w366:errorcluster)  [unwired: 11 in, 2 out]
            n188 = call "CallVI.vi"("VI引用"=w367, "状态"=T2."Hidden", "错误输入"=w366) -> ()  [unwired: 10 in, 3 out]
          }
          frame #1 {
            w376 = 0
            n189 = shared-variable "我的电脑\\Global.lvlib\\总成追溯码"("   " ("工位追溯码")) -> ()  [unwired: 1 in, 1 out]
            n190 = global write "Global.vi" "生产数量"(w376) -> ()
            n191 = global write "Global.vi" "合格数量"(w376) -> ()
            n192 = global read "Global1.vi" "用户信息"() -> (w371:T5)
            n193 = global read "Global1.vi" "联机模式"() -> (w370:enum16{"单机", "追溯"})
            n194 = Unbundle By Name(w371) -> ("用户名"=→"userName":string, "用户权限"=→"userStatus":string)
            n195 = case shown="\"追溯\"" w370 {
              tunnel: ["联网" ("connectionMode") "单机" ("connectionMode")] -> w377
              frame "追溯" {
              }
              frame "单机", Default {
              }
            }
            "connectionMode" <- w377
            "产品型号" <- "" ("产品型号")
          }
          frame #2 {
            n196 = control-ref of="表格控件"() -> (w382:refnum<vi>)
            n197 = control-ref of="提示信息"() -> (w384:refnum<vi>)
            n198 = control-ref of="自动"() -> (w385:refnum<vi>)
            n199 = control-ref of="错误"() -> (w386:refnum<vi>)
            n200 = control-ref of="更换产品"() -> (w383:refnum<vi>)
            n201 = global write "Global.vi" "提示信息"(w384) -> ()
            n202 = global write "Global.vi" "程序自动"(w385) -> ()
            n203 = global write "Global.vi" "报警图标"(w386) -> ()
            n204 = global write "Global.vi" "Result"(w382) -> ()
            n205 = global write "Global.vi" "更换产品"(w383) -> ()
            n206 = control-ref of="表格控件 2"() -> (w380:refnum<vi>)
            n207 = global write "Global.vi" "Result  右工位"(w380) -> ()
            n208 = control-ref of="上序状态"() -> (w381:refnum<vi>)
            n209 = global write "Global.vi" "上序状态"(w381) -> ()
          }
          frame #3 {
            w387 = -2
            n210 = global read "Global.vi" "Result"() -> (w390:refnum<vi>)
            n211 = property class="Tbl"(reference=w390, "Row Headers[]"=string[] [], "Value"=string[][] []) -> ()  [unwired: 1 in, 2 out]
            n212 = Bundle(w387, w387) -> (w388:cluster{i32, i32})  [unwired: 1 in]
            n213 = call "Start_Client.vi"() -> ()  [unwired: 12 in]
            n214 = property class="Tbl"(reference=w390, "Active Cell"=w388, "Cell BG Color"=u32 16777216 ("活动单元格:单元格背景色")) -> ()  [unwired: 1 in, 2 out]
          }
        }
        n215 = call <vilib>:"Add State(s) to Queue__jki_lib_state_machine.vi"("State(s) in (\"\")"=w363) -> ("States Out"=w362:string)  [unwired: 14 in]
      }
      frame "UI: Config" {
        n216 = vi-ref "Config.vi"() -> (w395:refnum<vi>)
        n217 = call "CallVI.vi"("VI引用"=w395, "状态"=T2."Standard") -> ()  [unwired: 11 in, 3 out]
        n218 = call <vilib>:"Add State(s) to Queue__jki_lib_state_machine.vi"("State(s) in (\"\")"=w400) -> ("States Out"=w399:string)  [unwired: 14 in]
      }
      frame "UI: Cursor Set" {
        # "Argument"
        n219 = case shown="\"Idle\", 默认" w403 {
          tunnel: w405 -> [w410 w412]
          tunnel: [w409 w411] -> w404
          frame "Idle", Default {
            n220 = call <vilib>:"Unset Busy.vi"("error in (no error)"=w410) -> ("error out"=w409:errorcluster)  [unwired: 10 in]
          }
          frame "Busy" {
            n221 = call <vilib>:"Set Busy.vi"("error in (no error)"=w412) -> ("error out"=w411:errorcluster)  [unwired: 9 in, 1 out]
          }
        }
        n222 = call <vilib>:"Add State(s) to Queue__jki_lib_state_machine.vi"("State(s) in (\"\")"=w408) -> ("States Out"=w407:string)  [unwired: 14 in]
      }
      frame "UI: Front Panel State" {
        # "Argument"
        n223 = Unbundle By Name(w417) -> ("Core.Current VI Reference"=w416:refnum<vi>)
        n224 = case shown="\"Close\"" w415 {
          tunnel: w419 -> [w425 w438]
          tunnel: [w427 w439] -> w418
          tunnel: w416 -> [w426 w436]
          frame "Open", Default {
            n225 = property class="VI"(reference=w426, error in=w425) -> (reference out=w423:refnum<vi>, error out=w424:errorcluster, "Front Panel.Open"=w422:bool)
            n226 = case shown="假" w422 {
              tunnel: [w430 w433] -> w427
              tunnel: w424 -> [w429 w433]
              tunnel: w423 -> [w428 _]
              frame False {
                n227 = invoke class="VI" method="FP.Open"(reference=w428, error in=w429, "Activate"=TRUE, "State"=T2."Standard") -> (error out=w430:errorcluster)  [unwired: 1 in, 4 out]
              }
              frame True {
              }
            }
          }
          frame "Close" {
            n228 = property class="VI"(reference=w436, error in=w438) -> (reference out=w435:refnum<vi>, error out=w437:errorcluster, "Front Panel.Open"=w434:bool)
            n229 = case shown="真" w434 {
              tunnel: [w440 w443] -> w439
              tunnel: w437 -> [w440 w442]
              tunnel: w435 -> [_ w441]
              frame False {
              }
              frame True {
                n230 = invoke class="VI" method="FP.Close"(reference=w441, error in=w442) -> (error out=w443:errorcluster)  [unwired: 1 in, 2 out]
              }
            }
          }
        }
        n231 = call <vilib>:"Add State(s) to Queue__jki_lib_state_machine.vi"("State(s) in (\"\")"=w421) -> ("States Out"=w420:string)  [unwired: 14 in]
      }
      frame "---------- Macro ----------" {
        n232 = call <vilib>:"Add State(s) to Queue__jki_lib_state_machine.vi"("State(s) in (\"\")"=w449) -> ("States Out"=w448:string)  [unwired: 14 in]
      }
      frame "Macro: Initialize" {
        n233 = call <vilib>:"Add State(s) to Queue__jki_lib_state_machine.vi"("State(s) in Front (\"\")"="Data: Initialize\nInitialize Core Data\nS7: Initialize\nIdle\nUI: Init\nUI: Front Panel State >> Open\nUI: Initialize\nUI: Config", "State(s) in (\"\")"=w456) -> ("States Out"=w455:string)  [unwired: 13 in]
      }
      frame "Macro: Exit" {
        n234 = Unbundle By Name(w465) -> ("Core.Close Panel on Exit?"=w464:bool)
        n235 = Select(t="UI: Front Panel State >> Close", s=w464, f="") -> (s? t:f=w461:string)
        n236 = call <vilib>:"Add State(s) to Queue__jki_lib_state_machine.vi"("State(s) in (\"\")"=w461, "State(s) at Back (\"\")"="Data: Cleanup\nExit") -> ("States Out"=w459:string)  [unwired: 13 in]
        n237 = call <vilib>:"Add State(s) to Queue__jki_lib_state_machine.vi"("State(s) in Front (\"\")"=w459, "State(s) in (\"\")"=w468) -> ("States Out"=w467:string)  [unwired: 13 in]
      }
    }
  }
  n238 = call-dynamic "Cleanup.vi"("MenuStrip in"=w6) -> ()  [unwired: 10 in, 1 out]
